vi "Dresden R2R Sputter 03.02.2018 IY24.vi"() -> ()   [LabVIEW 2009] (continued)
                                }
                                }
                                }
                                frame #1 {
                                }
                                }
                                }
                                frame #5 {
                                n16520 = local read "Semi"() -> (w26778:bool)
                                n16521 = case shown="False" w26778 {
                                frame #0 {
                                n16522 = while {
                                i -> [w26784]
                                stop <- w26780 stop-if-true
                                n16523 = local read "Tp1_stopped"() -> (w26782:bool)
                                n16524 = Greater?(x=w26784, y=120) -> (0:w26783:bool)
                                n16525 = local read "Semi"() -> (w26781:bool)
                                n16526 = Compound Arithmetic op=OR(w26781, w26782, w26783) -> (w26780:bool)
                                n16527 = Wait (ms)(milliseconds to wait=u32 500) -> ()  [unwired: 1 out]
                                }
                                }
                                frame #1 {
                                }
                                }
                                }
                                frame #6 {
                                n16528 = local read "Semi"() -> (w26786:bool)
                                n16529 = case shown="False" w26786 {
                                frame #0 {
                                n16530 = local read "Tp1_stopped"() -> (w26787:bool)
                                n16531 = case shown="False" w26787 {
                                frame #0 {
                                n16532 = local write "Error Message"("Shut Down process  cancelled\nbecause  TP not stopped.\nPlease check TP1 connections." ("Error Message")) -> ()
                                n16533 = local write "Semi"(TRUE ("Semi")) -> ()
                                }
                                frame #1 {
                                }
                                }
                                }
                                frame #1 {
                                }
                                }
                                }
                                }
                                }
                                frame #1 {
                                }
                                }
                                }
                                frame #1 {
                                n16534 = local read "Semi"() -> (w26790:bool)
                                n16535 = case shown="False" w26790 {
                                frame #0 {
                                n16536 = local write "Ch1_Sd0"(TRUE ("Ch1_Sd0")) -> ()
                                n16537 = Wait (ms)(milliseconds to wait=u32 1000) -> ()  [unwired: 1 out]
                                }
                                frame #1 {
                                }
                                }
                                }
                                }
                                }
                                frame #1 {
                                }
                                }
                              }
                              frame #2 {
                                # "CLOSE CC"
                                n16538 = local read "Semi"() -> (w26793:bool)
                                n16539 = case shown="False" w26793 {
                                frame #0 {
                                n16540 = stacked-sequence {
                                frame #0 {
                                n16541 = local read "Semi"() -> (w26794:bool)
                                n16542 = case shown="False" w26794 {
                                frame #0 {
                                n16543 = while {
                                i -> [w26800]
                                stop <- w26795 stop-if-true
                                n16544 = Greater?(x=w26800, y=25) -> (0:w26799:bool)
                                n16545 = case shown="True" w26799 {
                                frame #0 {
                                }
                                frame #1 {
                                n16546 = local write "Error Message"("Shut Down Process  cancelled\nbecause  CC not closed.\nPlease check CH1-CC connections." ("Error Message")) -> ()
                                n16547 = local write "Semi"(TRUE ("Semi")) -> ()
                                }
                                }
                                n16548 = local read "Ch1_Cc_on_off_di"() -> (w26798:bool)
                                n16549 = case shown="True" w26798 {
                                tunnel: [TRUE FALSE] -> w26796
                                frame #0 {
                                }
                                frame #1 {
                                n16550 = local write "Ch1_Cc_on_off_do"(FALSE ("Ch1_Ch_cc_on_off_di")) -> ()
                                n16551 = Wait Until Next ms Multiple(millisecond multiple=u32 200) -> ()  [unwired: 1 out]
                                }
                                }
                                n16552 = local read "Semi"() -> (w26797:bool)
                                n16553 = Or(x=w26796, y=w26797) -> (x .or. y?=w26795:bool)
                                }
                                }
                                frame #1 {
                                }
                                }
                                }
                                frame #1 {
                                n16554 = local read "Semi"() -> (w26808:bool)
                                n16555 = case shown="False" w26808 {
                                frame #0 {
                                n16556 = local write "Ch1_Sd1"(TRUE ("Ch1_Sd1")) -> ()
                                n16557 = Wait (ms)(milliseconds to wait=u32 1000) -> ()  [unwired: 1 out]
                                }
                                frame #1 {
                                }
                                }
                                }
                                }
                                }
                                frame #1 {
                                }
                                }
                              }
                              frame #3 {
                                # "CLOSE BG-BV"
                                n16558 = local read "Semi"() -> (w26811:bool)
                                n16559 = case shown="False" w26811 {
                                frame #0 {
                                n16560 = stacked-sequence {
                                frame #0 {
                                n16561 = local read "Semi"() -> (w26812:bool)
                                n16562 = case shown="False" w26812 {
                                frame #0 {
                                n16563 = while {
                                i -> [w26818]
                                stop <- w26813 stop-if-true
                                n16564 = Greater?(x=w26818, y=25) -> (0:w26817:bool)
                                n16565 = case shown="True" w26817 {
                                frame #0 {
                                }
                                frame #1 {
                                n16566 = local write "Error Message"("Shut Down Process  cancelled\nbecause  BG-BV not closed.\nPlease check BG-BV1 connections." ("Error Message")) -> ()
                                n16567 = local write "Semi"(TRUE ("Semi")) -> ()
                                }
                                }
                                n16568 = local read "Ch1_Bg_bv_di"() -> (w26816:bool)
                                n16569 = case shown="True" w26816 {
                                tunnel: [TRUE FALSE] -> w26814
                                frame #0 {
                                }
                                frame #1 {
                                n16570 = Wait Until Next ms Multiple(millisecond multiple=u32 200) -> ()  [unwired: 1 out]
                                n16571 = local write "Ch1_Bg_bv_do"(FALSE ("Ch1_Ch_cc_on_off_di")) -> ()
                                }
                                }
                                n16572 = local read "Semi"() -> (w26815:bool)
                                n16573 = Or(x=w26814, y=w26815) -> (x .or. y?=w26813:bool)
                                }
                                }
                                frame #1 {
                                }
                                }
                                }
                                frame #1 {
                                n16574 = local read "Semi"() -> (w26826:bool)
                                n16575 = case shown="False" w26826 {
                                frame #0 {
                                n16576 = Wait (ms)(milliseconds to wait=u32 1000) -> ()  [unwired: 1 out]
                                n16577 = local write "Ch1_Sd2"(TRUE ("Ch1_Sd1 2")) -> ()
                                }
                                frame #1 {
                                }
                                }
                                }
                                }
                                }
                                frame #1 {
                                }
                                }
                              }
                              frame #4 {
                                n16578 = local read "Yes"() -> (w26829:bool)
                                n16579 = case shown="True" w26829 {
                                frame #0 {
                                # "CLOSE PC-BV"
                                n16580 = local read "Semi"() -> (w26830:bool)
                                n16581 = case shown="False" w26830 {
                                frame #0 {
                                n16582 = stacked-sequence {
                                frame #0 {
                                n16583 = local read "Semi"() -> (w26831:bool)
                                n16584 = case shown="False" w26831 {
                                frame #0 {
                                n16585 = stacked-sequence {
                                frame #0 {
                                n16586 = local read "Semi"() -> (w26832:bool)
                                n16587 = case shown="False" w26832 {
                                frame #0 {
                                n16588 = local write "Pc_bv1_auto_close"(TRUE ("Tp1_auto_start")) -> ()
                                }
                                frame #1 {
                                }
                                }
                                }
                                frame #1 {
                                n16589 = local read "Semi"() -> (w26834:bool)
                                n16590 = case shown="False" w26834 {
                                frame #0 {
                                n16591 = Wait (ms)(milliseconds to wait=u32 1000) -> ()  [unwired: 1 out]
                                }
                                frame #1 {
                                }
                                }
                                }
                                frame #2 {
                                n16592 = local read "Semi"() -> (w26836:bool)
                                n16593 = case shown="False" w26836 {
                                frame #0 {
                                n16594 = while {
                                i -> [w26842]
                                stop <- w26838 stop-if-true
                                n16595 = local read "Pc_bv_closed_ch1"() -> (w26840:bool)
                                n16596 = Greater?(x=w26842, y=120) -> (0:w26841:bool)
                                n16597 = local read "Semi"() -> (w26839:bool)
                                n16598 = Compound Arithmetic op=OR(w26839, w26840, w26841) -> (w26838:bool)
                                n16599 = Wait (ms)(milliseconds to wait=u32 500) -> ()  [unwired: 1 out]
                                }
                                }
                                frame #1 {
                                }
                                }
                                }
                                frame #3 {
                                n16600 = local read "Semi"() -> (w26844:bool)
                                n16601 = case shown="False" w26844 {
                                frame #0 {
                                n16602 = local read "Pc_bv_closed_ch1"() -> (w26845:bool)
                                n16603 = case shown="False" w26845 {
                                frame #0 {
                                n16604 = local write "Pc_bv1_auto_close"(TRUE ("Pc_bv1_auto_open")) -> ()
                                }
                                frame #1 {
                                }
                                }
                                }
                                frame #1 {
                                }
                                }
                                }
                                frame #4 {
                                n16605 = local read "Semi"() -> (w26847:bool)
                                n16606 = case shown="False" w26847 {
                                frame #0 {
                                n16607 = local read "Pc_bv_closed_ch1"() -> (w26848:bool)
                                n16608 = case shown="False" w26848 {
                                frame #0 {
                                n16609 = Wait (ms)(milliseconds to wait=u32 1000) -> ()  [unwired: 1 out]
                                }
                                frame #1 {
                                }
                                }
                                }
                                frame #1 {
                                }
                                }
                                }
                                frame #5 {
                                n16610 = local read "Semi"() -> (w26850:bool)
                                n16611 = case shown="False" w26850 {
                                frame #0 {
                                n16612 = while {
                                i -> [w26856]
                                stop <- w26852 stop-if-true
                                n16613 = local read "Pc_bv_closed_ch1"() -> (w26854:bool)
                                n16614 = Greater?(x=w26856, y=120) -> (0:w26855:bool)
                                n16615 = local read "Semi"() -> (w26853:bool)
                                n16616 = Compound Arithmetic op=OR(w26853, w26854, w26855) -> (w26852:bool)
                                n16617 = Wait (ms)(milliseconds to wait=u32 500) -> ()  [unwired: 1 out]
                                }
                                }
                                frame #1 {
                                }
                                }
                                }
                                frame #6 {
                                n16618 = local read "Semi"() -> (w26858:bool)
                                n16619 = case shown="False" w26858 {
                                frame #0 {
                                n16620 = local read "Pc_bv_closed_ch1"() -> (w26859:bool)
                                n16621 = case shown="False" w26859 {
                                frame #0 {
                                n16622 = local write "Error Message"("Shut Down process  cancelled\nbecause  PC-BV not opened.\nPlease check PC-BV1 connections." ("Error Message")) -> ()
                                n16623 = local write "Semi"(TRUE ("Semi")) -> ()
                                }
                                frame #1 {
                                }
                                }
                                }
                                frame #1 {
                                }
                                }
                                }
                                }
                                }
                                frame #1 {
                                }
                                }
                                }
                                frame #1 {
                                n16624 = local read "Semi"() -> (w26862:bool)
                                n16625 = case shown="False" w26862 {
                                frame #0 {
                                n16626 = Wait (ms)(milliseconds to wait=u32 1000) -> ()  [unwired: 1 out]
                                n16627 = local write "Ch1_Sd3"(TRUE ("Ch1_Sd2")) -> ()
                                }
                                frame #1 {
                                }
                                }
                                }
                                }
                                }
                                frame #1 {
                                }
                                }
                                }
                                frame #1 {
                                # "OPEN PC-BV"
                                n16628 = local read "Semi"() -> (w26865:bool)
                                n16629 = case shown="False" w26865 {
                                frame #0 {
                                n16630 = stacked-sequence {
                                frame #0 {
                                n16631 = local read "Semi"() -> (w26866:bool)
                                n16632 = case shown="False" w26866 {
                                frame #0 {
                                n16633 = stacked-sequence {
                                frame #0 {
                                n16634 = local read "Semi"() -> (w26867:bool)
                                n16635 = case shown="False" w26867 {
                                frame #0 {
                                n16636 = local write "Pc_bv1_auto_open"(TRUE ("Tp1_auto_start")) -> ()
                                }
                                frame #1 {
                                }
                                }
                                }
                                frame #1 {
                                n16637 = local read "Semi"() -> (w26869:bool)
                                n16638 = case shown="False" w26869 {
                                frame #0 {
                                n16639 = Wait (ms)(milliseconds to wait=u32 1000) -> ()  [unwired: 1 out]
                                }
                                frame #1 {
                                }
                                }
                                }
                                frame #2 {
                                n16640 = local read "Semi"() -> (w26871:bool)
                                n16641 = case shown="False" w26871 {
                                frame #0 {
                                n16642 = while {
                                i -> [w26877]
                                stop <- w26873 stop-if-true
                                n16643 = local read "Pc_bv_opened_ch1"() -> (w26875:bool)
                                n16644 = Greater?(x=w26877, y=120) -> (0:w26876:bool)
                                n16645 = local read "Semi"() -> (w26874:bool)
                                n16646 = Compound Arithmetic op=OR(w26874, w26875, w26876) -> (w26873:bool)
                                n16647 = Wait (ms)(milliseconds to wait=u32 500) -> ()  [unwired: 1 out]
                                }
                                }
                                frame #1 {
                                }
                                }
                                }
                                frame #3 {
                                n16648 = local read "Semi"() -> (w26879:bool)
                                n16649 = case shown="False" w26879 {
                                frame #0 {
                                n16650 = local read "Pc_bv_opened_ch1"() -> (w26880:bool)
                                n16651 = case shown="False" w26880 {
                                frame #0 {
                                n16652 = local write "Pc_bv1_auto_open"(TRUE ("Pc_bv1_auto_open")) -> ()
                                }
                                frame #1 {
                                }
                                }
                                }
                                frame #1 {
                                }
                                }
                                }
                                frame #4 {
                                n16653 = local read "Semi"() -> (w26882:bool)
                                n16654 = case shown="False" w26882 {
                                frame #0 {
                                n16655 = local read "Pc_bv_opened_ch1"() -> (w26883:bool)
                                n16656 = case shown="False" w26883 {
                                frame #0 {
                                n16657 = Wait (ms)(milliseconds to wait=u32 1000) -> ()  [unwired: 1 out]
                                }
                                frame #1 {
                                }
                                }
                                }
                                frame #1 {
                                }
                                }
                                }
                                frame #5 {
                                n16658 = local read "Semi"() -> (w26885:bool)
                                n16659 = case shown="False" w26885 {
                                frame #0 {
                                n16660 = while {
                                i -> [w26891]
                                stop <- w26887 stop-if-true
                                n16661 = local read "Pc_bv_opened_ch1"() -> (w26889:bool)
                                n16662 = Greater?(x=w26891, y=120) -> (0:w26890:bool)
                                n16663 = local read "Semi"() -> (w26888:bool)
                                n16664 = Compound Arithmetic op=OR(w26888, w26889, w26890) -> (w26887:bool)
                                n16665 = Wait (ms)(milliseconds to wait=u32 500) -> ()  [unwired: 1 out]
                                }
                                }
                                frame #1 {
                                }
                                }
                                }
                                frame #6 {
                                n16666 = local read "Semi"() -> (w26893:bool)
                                n16667 = case shown="False" w26893 {
                                frame #0 {
                                n16668 = local read "Pc_bv_opened_ch1"() -> (w26894:bool)
                                n16669 = case shown="False" w26894 {
                                frame #0 {
                                n16670 = local write "Error Message"("Shut Down process  cancelled\nbecause  PC-BV not opened.\nPlease check PC-BV1 connections." ("Error Message")) -> ()
                                n16671 = Wait (ms)(milliseconds to wait=u32 1000) -> ()  [unwired: 1 out]
                                }
                                frame #1 {
                                }
                                }
                                }
                                frame #1 {
                                }
                                }
                                }
                                }
                                }
                                frame #1 {
                                }
                                }
                                }
                                frame #1 {
                                n16672 = local read "Semi"() -> (w26897:bool)
                                n16673 = case shown="False" w26897 {
                                frame #0 {
                                n16674 = Wait (ms)(milliseconds to wait=u32 1000) -> ()  [unwired: 1 out]
                                n16675 = local write "Ch1_Sd4"(TRUE ("Ch1_Sd2")) -> ()
                                }
                                frame #1 {
                                }
                                }
                                }
                                }
                                }
                                frame #1 {
                                }
                                }
                                }
                                }
                              }
                              frame #5 {
                                # "CLOSE TP-BV"
                                n16676 = local read "Semi"() -> (w26900:bool)
                                n16677 = case shown="False" w26900 {
                                frame #0 {
                                n16678 = stacked-sequence {
                                frame #0 {
                                n16679 = local read "Semi"() -> (w26901:bool)
                                n16680 = case shown="False" w26901 {
                                frame #0 {
                                n16681 = while {
                                i -> [w26907]
                                stop <- w26902 stop-if-true
                                n16682 = Greater?(x=w26907, y=25) -> (0:w26906:bool)
                                n16683 = case shown="True" w26906 {
                                frame #0 {
                                }
                                frame #1 {
                                n16684 = local write "Error Message"("Shut Down Process  cancelled\nbecause  TP-BV not closed.\nPlease check TP-BV1 connections." ("Error Message")) -> ()
                                n16685 = local write "Semi"(TRUE ("Semi")) -> ()
                                }
                                }
                                n16686 = local read "Ch1_Tp_bv_di"() -> (w26905:bool)
                                n16687 = case shown="True" w26905 {
                                tunnel: [TRUE FALSE] -> w26903
                                frame #0 {
                                }
                                frame #1 {
                                n16688 = Wait Until Next ms Multiple(millisecond multiple=u32 200) -> ()  [unwired: 1 out]
                                n16689 = local write "Ch1_Tp_bv_do"(FALSE ("Ch1_Ch_cc_on_off_di")) -> ()
                                }
                                }
                                n16690 = local read "Semi"() -> (w26904:bool)
                                n16691 = Or(x=w26903, y=w26904) -> (x .or. y?=w26902:bool)
                                }
                                }
                                frame #1 {
                                }
                                }
                                }
                                frame #1 {
                                n16692 = local read "Semi"() -> (w26915:bool)
                                n16693 = case shown="False" w26915 {
                                frame #0 {
                                n16694 = local write "Ch1_Sd5"(TRUE ("Ch1_Sd5")) -> ()
                                n16695 = Wait (ms)(milliseconds to wait=u32 1000) -> ()  [unwired: 1 out]
                                }
                                frame #1 {
                                }
                                }
                                }
                                }
                                }
                                frame #1 {
                                }
                                }
                              }
                              frame #6 {
                                # "STOP MP"
                                n16696 = local read "Semi"() -> (w26918:bool)
                                n16697 = case shown="False" w26918 {
                                frame #0 {
                                n16698 = stacked-sequence {
                                frame #0 {
                                n16699 = local read "Semi"() -> (w26919:bool)
                                n16700 = case shown="False" w26919 {
                                frame #0 {
                                n16701 = while {
                                i -> [w26925]
                                stop <- w26920 stop-if-true
                                n16702 = Greater?(x=w26925, y=25) -> (0:w26924:bool)
                                n16703 = case shown="True" w26924 {
                                frame #0 {
                                }
                                frame #1 {
                                n16704 = local write "Error Message"("Shut Down Process  cancelled\nbecause  MP not closed.\nPlease check MP1 connections." ("Error Message")) -> ()
                                n16705 = local write "Semi"(TRUE ("Semi")) -> ()
                                }
                                }
                                n16706 = local read "Ch1_Mp_di"() -> (w26923:bool)
                                n16707 = case shown="True" w26923 {
                                tunnel: [TRUE FALSE] -> w26921
                                frame #0 {
                                }
                                frame #1 {
                                n16708 = Wait Until Next ms Multiple(millisecond multiple=u32 200) -> ()  [unwired: 1 out]
                                n16709 = local write "Ch1_Mp_do"(FALSE ("Ch1_Ch_cc_on_off_di")) -> ()
                                }
                                }
                                n16710 = local read "Semi"() -> (w26922:bool)
                                n16711 = Or(x=w26921, y=w26922) -> (x .or. y?=w26920:bool)
                                }
                                }
                                frame #1 {
                                }
                                }
                                }
                                frame #1 {
                                n16712 = local read "Semi"() -> (w26933:bool)
                                n16713 = case shown="False" w26933 {
                                frame #0 {
                                n16714 = local write "Ch1_Sd6"(TRUE ("Ch1_Sd6")) -> ()
                                n16715 = Wait (ms)(milliseconds to wait=u32 1000) -> ()  [unwired: 1 out]
                                }
                                frame #1 {
                                }
                                }
                                }
                                }
                                }
                                frame #1 {
                                }
                                }
                              }
                              frame #7 {
                                # "PL-VBV OPEN  & CHECK"
                                n16716 = local read "Semi"() -> (w26936:bool)
                                n16717 = case shown="False" w26936 {
                                frame #0 {
                                n16718 = stacked-sequence {
                                frame #0 {
                                n16719 = local read "Semi"() -> (w26937:bool)
                                n16720 = case shown="False" w26937 {
                                frame #0 {
                                n16721 = local write "Ch1_Pl_atm_do"(FALSE ("Ch1_Pl_atm_do")) -> ()
                                n16722 = Wait Until Next ms Multiple(millisecond multiple=u32 2000) -> ()  [unwired: 1 out]
                                }
                                frame #1 {
                                }
                                }
                                }
                                frame #1 {
                                n16723 = local read "Semi"() -> (w26940:bool)
                                n16724 = case shown="False" w26940 {
                                frame #0 {
                                n16725 = while {
                                i -> [w26946]
                                stop <- w26942 stop-if-true
                                n16726 = Greater?(x=w26946, y=50) -> (0:w26945:bool)
                                n16727 = case shown="True" w26945 {
                                frame #0 {
                                }
                                frame #1 {
                                n16728 = local write "Error Message"("Shut Down Process  cancelled\nbecause  PL-VBV not opened.\nPlease check  PL-VBV1 connections." ("Error Message")) -> ()
                                n16729 = local write "Semi"(TRUE ("Semi")) -> ()
                                }
                                }
                                n16730 = local read "Ch1_Pl_atm_di"() -> (w26941:bool)
                                n16731 = case shown="False" w26941 {
                                tunnel: [w26948 TRUE] -> w26943
                                frame #0 {
                                n16732 = local read "Ch1_Pl_vbv_di"() -> (w26949:bool)
                                n16733 = case shown="False" w26949 {
                                tunnel: [FALSE TRUE] -> w26948
                                frame #0 {
                                n16734 = Wait Until Next ms Multiple(millisecond multiple=u32 500) -> ()  [unwired: 1 out]
                                n16735 = local write "Ch1_Pl_vbv_do"(TRUE ("Ch1_Ch_cc_on_off_di")) -> ()
                                }
                                frame #1 {
                                }
                                }
                                }
                                frame #1 {
                                n16736 = Wait Until Next ms Multiple(millisecond multiple=u32 500) -> ()  [unwired: 1 out]
                                }
                                }
                                n16737 = local read "Semi"() -> (w26944:bool)
                                n16738 = Or(x=w26943, y=w26944) -> (x .or. y?=w26942:bool)
                                }
                                }
                                frame #1 {
                                }
                                }
                                }
                                frame #2 {
                                n16739 = local read "Semi"() -> (w26958:bool)
                                n16740 = case shown="False" w26958 {
                                frame #0 {
                                n16741 = local write "Ch1_Sd7"(FALSE ("Ch1_Sd8")) -> ()
                                n16742 = Wait (ms)(milliseconds to wait=u32 1000) -> ()  [unwired: 1 out]
                                }
                                frame #1 {
                                }
                                }
                                }
                                }
                                }
                                frame #1 {
                                }
                                }
                              }
                              frame #8 {
                                # "PL-VBV CLOSE  & CHECK"
                                n16743 = local read "Semi"() -> (w26961:bool)
                                n16744 = case shown="False" w26961 {
                                frame #0 {
                                n16745 = stacked-sequence {
                                frame #0 {
                                n16746 = local read "Semi"() -> (w26962:bool)
                                n16747 = case shown="False" w26962 {
                                frame #0 {
                                n16748 = while {
                                i -> [w26968]
                                stop <- w26964 stop-if-true
                                n16749 = Greater?(x=w26968, y=50) -> (0:w26967:bool)
                                n16750 = case shown="True" w26967 {
                                frame #0 {
                                }
                                frame #1 {
                                n16751 = local write "Error Message"("Shut Down Process  cancelled\nbecause  PL-VBV not closed.\nPlease check PL-VBV1 connections." ("Error Message")) -> ()
                                n16752 = local write "Semi"(TRUE ("Semi")) -> ()
                                }
                                }
                                n16753 = local read "Ch1_Pl_atm_di"() -> (w26963:bool)
                                n16754 = case shown="True" w26963 {
                                tunnel: [FALSE w26972] -> w26965
                                frame #0 {
                                n16755 = Wait Until Next ms Multiple(millisecond multiple=u32 500) -> ()  [unwired: 1 out]
                                }
                                frame #1 {
                                n16756 = local read "Ch1_Pl_vbv_di"() -> (w26973:bool)
                                n16757 = case shown="True" w26973 {
                                tunnel: [TRUE FALSE] -> w26972
                                frame #0 {
                                }
                                frame #1 {
                                n16758 = Wait Until Next ms Multiple(millisecond multiple=u32 500) -> ()  [unwired: 1 out]
                                n16759 = local write "Ch1_Pl_vbv_do"(FALSE ("Ch1_Ch_cc_on_off_di")) -> ()
                                }
                                }
                                }
                                }
                                n16760 = local read "Semi"() -> (w26966:bool)
                                n16761 = Or(x=w26965, y=w26966) -> (x .or. y?=w26964:bool)
                                }
                                }
                                frame #1 {
                                }
                                }
                                }
                                frame #1 {
                                n16762 = local read "Semi"() -> (w26980:bool)
                                n16763 = case shown="False" w26980 {
                                frame #0 {
                                n16764 = local write "Ch1_Sd8"(TRUE ("Ch1_Sd11")) -> ()
                                n16765 = Wait (ms)(milliseconds to wait=u32 1000) -> ()  [unwired: 1 out]
                                }
                                frame #1 {
                                }
                                }
                                }
                                }
                                }
                                frame #1 {
                                }
                                }
                              }
                              frame #9 {
                                # "WAIT DECELARATING TP"
                                n16766 = local read "Semi"() -> (w26983:bool)
                                n16767 = case shown="False" w26983 {
                                frame #0 {
                                n16768 = stacked-sequence {
                                frame #0 {
                                n16769 = local read "Semi"() -> (w26984:bool)
                                n16770 = case shown="False" w26984 {
                                frame #0 {
                                n16771 = while {
                                i -> [w26990]
                                stop <- w26986 stop-if-true
                                n16772 = Greater?(x=w26990, y=1500) -> (0:w26989:bool)
                                n16773 = case shown="True" w26989 {
                                frame #0 {
                                }
                                frame #1 {
                                n16774 = local write "Error Message"("Shut Down Process  cancelled\nbecause TP not decelarating.\nPlease check TP1 connections." ("Error Message")) -> ()
                                n16775 = local write "Semi"(TRUE ("Semi")) -> ()
                                }
                                }
                                n16776 = local read "Yes"() -> (w26985:bool)
                                n16777 = case shown="True" w26985 {
                                tunnel: [TRUE w26996] -> w26987
                                frame #0 {
                                }
                                frame #1 {
                                n16778 = local read "Tp1_speed_gui"() -> (w26994:i32)
                                n16779 = Less?(x=w26994, y="Tp1_safety_speed") -> (x < y?=w26993:bool)
                                n16780 = case shown="False" w26993 {
                                tunnel: [FALSE TRUE] -> w26996
                                frame #0 {
                                n16781 = Wait Until Next ms Multiple(millisecond multiple=u32 500) -> ()  [unwired: 1 out]
                                }
                                frame #1 {
                                }
                                }
                                }
                                }
                                n16782 = local read "Semi"() -> (w26988:bool)
                                n16783 = Or(x=w26987, y=w26988) -> (x .or. y?=w26986:bool)
                                }
                                }
                                frame #1 {
                                }
                                }
                                }
                                frame #1 {
                                n16784 = local read "Semi"() -> (w27002:bool)
                                n16785 = case shown="False" w27002 {
                                frame #0 {
                                n16786 = Wait (ms)(milliseconds to wait=u32 1000) -> ()  [unwired: 1 out]
                                n16787 = local write "Ch1_Sd9"(TRUE ("Ch1_Sd3")) -> ()
                                }
                                frame #1 {
                                }
                                }
                                }
                                }
                                }
                                frame #1 {
                                }
                                }
                              }
                              frame #10 {
                                # "CH-VBV OPEN  & CHECK"
                                n16788 = local read "Yes"() -> (w27005:bool)
                                n16789 = case shown="True" w27005 {
                                frame #0 {
                                }
                                frame #1 {
                                n16790 = local read "Semi"() -> (w27006:bool)
                                n16791 = case shown="False" w27006 {
                                frame #0 {
                                n16792 = stacked-sequence {
                                frame #0 {
                                n16793 = local read "Semi"() -> (w27007:bool)
                                n16794 = case shown="False" w27007 {
                                frame #0 {
                                n16795 = local write "Ch1_Ch_atm_do"(FALSE ("Ch1_Pl_atm_do")) -> ()
                                n16796 = Wait Until Next ms Multiple(millisecond multiple=u32 2000) -> ()  [unwired: 1 out]
                                }
                                frame #1 {
                                }
                                }
                                }
                                frame #1 {
                                n16797 = local read "Semi"() -> (w27010:bool)
                                n16798 = case shown="False" w27010 {
                                frame #0 {
                                n16799 = while {
                                i -> [w27016]
                                stop <- w27012 stop-if-true
                                n16800 = Greater?(x=w27016, y=50) -> (0:w27015:bool)
                                n16801 = case shown="True" w27015 {
                                frame #0 {
                                }
                                frame #1 {
                                n16802 = local write "Error Message"("Shut Down Process  cancelled\nbecause  CH-VBV not opened.\nPlease check  CH-VBV1 connections." ("Error Message")) -> ()